vi "Dresden R2R Sputter 03.02.2018 IY24.vi"() -> ()   [LabVIEW 2009] (continued)
                                n30013 = Wait Until Next ms Multiple(millisecond multiple=u32 200) -> ()  [unwired: 1 out]
                                }
                                }
                                n30014 = local read "Semi"() -> (w34901:bool)
                                n30015 = Or(x=w34902, y=w34901) -> (x .or. y?=w34900:bool)
                                }
                                }
                                frame #1 {
                                }
                                }
                                }
                                frame #1 {
                                n30016 = local read "Semi"() -> (w34913:bool)
                                n30017 = case shown="False" w34913 {
                                frame #0 {
                                n30018 = local write "SDC1 10b"(TRUE ("SDC1 3")) -> ()
                                n30019 = Wait (ms)(milliseconds to wait=u32 1000) -> ()  [unwired: 1 out]
                                }
                                frame #1 {
                                }
                                }
                                }
                                }
                                }
                                frame #12 {
                                # "DC -Ignite Plasma"
                                n30020 = stacked-sequence {
                                frame #0 {
                                n30021 = local read "Semi"() -> (w34916:bool)
                                n30022 = case shown="False" w34916 {
                                frame #0 {
                                n30023 = stacked-sequence {
                                frame #0 {
                                n30024 = local read "Semi"() -> (w34917:bool)
                                n30025 = case shown="False" w34917 {
                                frame #0 {
                                n30026 = while {
                                i -> [w34923]
                                stop <- w34918 stop-if-true
                                n30027 = Greater?(x=w34923, y=50) -> (0:w34922:bool)
                                n30028 = case shown="True" w34922 {
                                frame #0 {
                                }
                                frame #1 {
                                n30029 = local write "Semi"(TRUE ("Semi")) -> ()
                                n30030 = local write "Error Message"("Sputtering Process cancelled.\nPlease check \nDC switch connections." ("Error Message")) -> ()
                                }
                                }
                                n30031 = local read "Cnt_Dcps_sw2_di"() -> (w34921:bool)
                                n30032 = case shown="False" w34921 {
                                tunnel: [FALSE ("Cnt_Dcps_sw1_do") TRUE ("Cnt_Dcps_sw1_do")] -> w34920
                                frame #0 {
                                n30033 = local write "Cnt_Dcps_sw2_do"(TRUE ("Cnt_Dcps_sw1_do")) -> ()
                                n30034 = Wait Until Next ms Multiple(millisecond multiple=u32 200) -> ()  [unwired: 1 out]
                                }
                                frame #1 {
                                }
                                }
                                n30035 = local read "Semi"() -> (w34919:bool)
                                n30036 = Or(x=w34920, y=w34919) -> (x .or. y?=w34918:bool)
                                }
                                }
                                frame #1 {
                                }
                                }
                                }
                                frame #1 {
                                n30037 = local read "Semi"() -> (w34931:bool)
                                n30038 = case shown="False" w34931 {
                                frame #0 {
                                n30039 = while {
                                i -> [w34937]
                                stop <- w34932 stop-if-true
                                n30040 = Greater?(x=w34937, y=50) -> (0:w34936:bool)
                                n30041 = case shown="True" w34936 {
                                frame #0 {
                                }
                                frame #1 {
                                n30042 = local write "Semi"(TRUE ("Semi")) -> ()
                                n30043 = local write "Error Message"("Sputtering Process cancelled.\nPlease check \nDC switch connections." ("Error Message")) -> ()
                                }
                                }
                                n30044 = local read "Cnt_Dcps_sw1_di"() -> (w34935:bool)
                                n30045 = case shown="True" w34935 {
                                tunnel: [TRUE ("Cnt_Dcps_sw1_do") FALSE ("Cnt_Dcps_sw1_do")] -> w34934
                                frame #0 {
                                }
                                frame #1 {
                                n30046 = local write "Cnt_Dcps_sw1_do"(FALSE ("Cnt_Dcps_sw1_do")) -> ()
                                n30047 = Wait Until Next ms Multiple(millisecond multiple=u32 200) -> ()  [unwired: 1 out]
                                }
                                }
                                n30048 = local read "Semi"() -> (w34933:bool)
                                n30049 = Or(x=w34934, y=w34933) -> (x .or. y?=w34932:bool)
                                }
                                }
                                frame #1 {
                                }
                                }
                                }
                                frame #2 {
                                n30050 = local read "Semi"() -> (w34945:bool)
                                n30051 = case shown="False" w34945 {
                                frame #0 {
                                n30052 = local write "Dc_host_auto"(TRUE ("Dc_host_auto")) -> ()
                                }
                                frame #1 {
                                }
                                }
                                }
                                frame #3 {
                                n30053 = local read "Semi"() -> (w34947:bool)
                                n30054 = case shown="False" w34947 {
                                frame #0 {
                                n30055 = local read "R Cmb Ch3 Step1 Coating Power"() -> (w34948:dbl)
                                n30056 = local write "Set DC Power       : 2"(w34948) -> ()
                                }
                                frame #1 {
                                }
                                }
                                }
                                frame #4 {
                                n30057 = local read "Semi"() -> (w34949:bool)
                                n30058 = case shown="False" w34949 {
                                frame #0 {
                                n30059 = Wait (ms)(milliseconds to wait=u32 1000) -> ()  [unwired: 1 out]
                                }
                                frame #1 {
                                }
                                }
                                }
                                frame #5 {
                                n30060 = local read "Semi"() -> (w34951:bool)
                                n30061 = case shown="False" w34951 {
                                frame #0 {
                                n30062 = local write "Dc_auto_set"(TRUE ("Dc_auto_set")) -> ()
                                }
                                frame #1 {
                                }
                                }
                                }
                                frame #6 {
                                n30063 = local read "Semi"() -> (w34953:bool)
                                n30064 = case shown="False" w34953 {
                                frame #0 {
                                n30065 = Wait (ms)(milliseconds to wait=u32 1000) -> ()  [unwired: 1 out]
                                }
                                frame #1 {
                                }
                                }
                                }
                                }
                                }
                                frame #1 {
                                }
                                }
                                }
                                frame #1 {
                                n30066 = local read "Semi"() -> (w34955:bool)
                                n30067 = case shown="False" w34955 {
                                frame #0 {
                                n30068 = Wait (ms)(milliseconds to wait=u32 1000) -> ()  [unwired: 1 out]
                                n30069 = local write "SDC1 13"(TRUE ("SDC1 13")) -> ()
                                }
                                frame #1 {
                                }
                                }
                                }
                                }
                                }
                                frame #13 {
                                n30070 = stacked-sequence {
                                frame #0 {
                                n30071 = local read "R Maximum diameter"() -> (w34959:dbl)
                                n30072 = local read "R Web speed(cm/min)"() -> (w34961:dbl)
                                n30073 = local read "R Minimum diameter"() -> (w34958:dbl)
                                n30074 = local read "R Web thicness"() -> (w34960:dbl)
                                n30075 = Wait (ms)(milliseconds to wait=u32 1000) -> ()  [unwired: 1 out]
                                n30076 = local write "Initial Min Diameter"(w34958) -> ()
                                n30077 = local write "Max Diameter"(w34959) -> ()
                                n30078 = local write "Web Thickness"(w34960) -> ()
                                n30079 = local write "Web Speed"(w34961) -> ()
                                }
                                frame #1 {
                                n30080 = local read "R Cmb Ch2 Step1 Coating Power Active"() -> (w34976:bool)
                                n30081 = local read "R Cmb Ch2 Step2 Coating Power Active"() -> (w34975:bool)
                                n30082 = local read "R Cmb Ch2 Step3 Coating Power Active"() -> (w34974:bool)
                                n30083 = local read "R Cmb Ch2 Step4 Coating Power Active"() -> (w34973:bool)
                                n30084 = local read "R Cmb Ch2 Step5 Coating Power Active"() -> (w34972:bool)
                                n30085 = Boolean To (0,1)(Boolean=w34976) -> (0, 1=w34971:i16)
                                n30086 = Boolean To (0,1)(Boolean=w34975) -> (0, 1=w34970:i16)
                                n30087 = Boolean To (0,1)(Boolean=w34974) -> (0, 1=w34969:i16)
                                n30088 = Boolean To (0,1)(Boolean=w34973) -> (0, 1=w34968:i16)
                                n30089 = Boolean To (0,1)(Boolean=w34972) -> (0, 1=w34967:i16)
                                n30090 = Compound Arithmetic op=ADD(w34971, w34970, w34969, w34968, w34967) -> (w34965:i16)
                                n30091 = local read "R Cmb Interval length"() -> (w34966:dbl)
                                n30092 = Wait (ms)(milliseconds to wait=u32 200) -> ()  [unwired: 1 out]
                                n30093 = Multiply(x=w34966, y=w34965) -> (x*y=w34964:dbl)
                                n30094 = local write "Total length"(w34964) -> ()
                                }
                                frame #2 {
                                n30095 = local write "Calculate 2"(TRUE ("Calculate_auto")) -> ()
                                }
                                frame #3 {
                                n30096 = Wait (ms)(milliseconds to wait=u32 100) -> ()  [unwired: 1 out]
                                n30097 = local write "Roll_side_select"(enum32{"Left to Right", "Right to Left"}."Left to Right" ("Roll_side_select")) -> ()
                                }
                                frame #4 {
                                n30098 = Wait (ms)(milliseconds to wait=u32 100) -> ()  [unwired: 1 out]
                                n30099 = local write "Parameters_auto_set"(TRUE ("Parameters_auto_set")) -> ()
                                }
                                frame #5 {
                                n30100 = while {
                                i -> [w34986]
                                stop <- w34982 stop-if-true
                                n30101 = Wait Until Next ms Multiple(millisecond multiple=u32 300) -> ()  [unwired: 1 out]
                                n30102 = Greater?(x=w34986, y=100) -> (0:w34983:bool)
                                n30103 = local read "Parameters_auto_set"() -> (w34987:bool)
                                n30104 = case shown="False" w34987 {
                                tunnel: [TRUE FALSE] -> w34984
                                frame #0 {
                                }
                                frame #1 {
                                }
                                }
                                n30105 = Or(x=w34984, y=w34983) -> (x .or. y?=w34982:bool)
                                }
                                }
                                frame #6 {
                                n30106 = local read "R Tension Value"() -> (w34991:dbl)
                                n30107 = Wait (ms)(milliseconds to wait=u32 200) -> ()  [unwired: 1 out]
                                n30108 = local write "TC1_set_value"(w34991) -> ()
                                }
                                frame #7 {
                                n30109 = local write "TC1_auto_set"(TRUE ("TC1_auto_set")) -> ()
                                }
                                frame #8 {
                                w34995 = u16 2 items=["1", "2", "3", "4"] ("Target Chamber Sensor")
                                n30110 = local write "Target Chamber Sensor"(w34995) -> ()
                                n30111 = Wait (ms)(milliseconds to wait=u32 200) -> ()  [unwired: 1 out]
                                }
                                frame #9 {
                                n30112 = local read "Total length"() -> (w34997:dbl)
                                n30113 = Wait (ms)(milliseconds to wait=u32 100) -> ()  [unwired: 1 out]
                                n30114 = local write "Region"(w34997) -> ()
                                }
                                frame #10 {
                                n30115 = local read "Semi"() -> (w34998:bool)
                                n30116 = case shown="False" w34998 {
                                frame #0 {
                                n30117 = stacked-sequence {
                                frame #0 {
                                # "Gas Flow"
                                n30118 = stacked-sequence {
                                frame #0 {
                                n30119 = local read "Semi"() -> (w34999:bool)
                                n30120 = case shown="False" w34999 {
                                frame #0 {
                                n30121 = stacked-sequence {
                                frame #0 {
                                n30122 = local read "Semi"() -> (w35000:bool)
                                n30123 = case shown="False" w35000 {
                                frame #0 {
                                n30124 = local read "R Argon Flow sccm"() -> (w35001:dbl)
                                n30125 = local write "Ar_sccm3_4"(w35001) -> ()
                                }
                                frame #1 {
                                }
                                }
                                }
                                frame #1 {
                                n30126 = local read "Semi"() -> (w35002:bool)
                                n30127 = case shown="False" w35002 {
                                frame #0 {
                                n30128 = local write "Mfc2_Ar _3_4_set"(TRUE ("Mfc_Ar _1_2_set")) -> ()
                                }
                                frame #1 {
                                }
                                }
                                }
                                frame #2 {
                                n30129 = local read "Semi"() -> (w35004:bool)
                                n30130 = case shown="False" w35004 {
                                frame #0 {
                                n30131 = while {
                                i -> [w35007]
                                stop <- w35009 stop-if-true
                                n30132 = Greater?(x=w35007, y=50) -> (0:w35006:bool)
                                n30133 = local read "Semi"() -> (w35005:bool)
                                n30134 = Or(x=w35005, y=w35006) -> (x .or. y?=w35009:bool)
                                }
                                }
                                frame #1 {
                                }
                                }
                                }
                                frame #3 {
                                n30135 = local read "Semi"() -> (w35010:bool)
                                n30136 = case shown="False" w35010 {
                                frame #0 {
                                n30137 = local read "Ar_sccm_act 2"() -> (w35011:dbl)
                                n30138 = Greater?(x=w35011, y=1) -> (0:w35012:bool)
                                n30139 = case shown="False" w35012 {
                                frame #0 {
                                n30140 = local read "R Argon Flow sccm"() -> (w35014:dbl)
                                n30141 = local write "Ar_sccm3_4"(w35014) -> ()
                                }
                                frame #1 {
                                }
                                }
                                }
                                frame #1 {
                                }
                                }
                                }
                                frame #4 {
                                n30142 = local read "Semi"() -> (w35015:bool)
                                n30143 = case shown="False" w35015 {
                                frame #0 {
                                n30144 = local read "Ar_sccm_act 2"() -> (w35016:dbl)
                                n30145 = Greater?(x=w35016, y=1) -> (0:w35017:bool)
                                n30146 = case shown="False" w35017 {
                                frame #0 {
                                n30147 = while {
                                i -> [w35020]
                                stop <- w35024 stop-if-true
                                n30148 = Greater?(x=w35020, y=50) -> (0:w35019:bool)
                                n30149 = local read "Semi"() -> (w35023:bool)
                                n30150 = case shown="False" w35023 {
                                tunnel: [FALSE TRUE] -> w35022
                                frame #0 {
                                n30151 = Wait Until Next ms Multiple(millisecond multiple=u32 200) -> ()  [unwired: 1 out]
                                }
                                frame #1 {
                                }
                                }
                                n30152 = Or(x=w35022, y=w35019) -> (x .or. y?=w35024:bool)
                                }
                                }
                                frame #1 {
                                }
                                }
                                }
                                frame #1 {
                                }
                                }
                                }
                                frame #5 {
                                n30153 = local read "Semi"() -> (w35028:bool)
                                n30154 = case shown="False" w35028 {
                                frame #0 {
                                n30155 = local read "Ar_sccm_act 2"() -> (w35029:dbl)
                                n30156 = Greater?(x=w35029, y=1) -> (0:w35030:bool)
                                n30157 = case shown="False" w35030 {
                                frame #0 {
                                n30158 = local write "Semi"(TRUE ("Semi")) -> ()
                                n30159 = local write "Error Message"("Coating process cancelled.\nPlease check connections." ("Error Message")) -> ()
                                }
                                frame #1 {
                                }
                                }
                                }
                                frame #1 {
                                }
                                }
                                }
                                }
                                }
                                frame #1 {
                                }
                                }
                                }
                                frame #1 {
                                n30160 = local read "Semi"() -> (w35034:bool)
                                n30161 = case shown="False" w35034 {
                                frame #0 {
                                n30162 = local write "SDC1 11"(TRUE ("SDC1 11")) -> ()
                                n30163 = Wait (ms)(milliseconds to wait=u32 1000) -> ()  [unwired: 1 out]
                                }
                                frame #1 {
                                }
                                }
                                }
                                }
                                }
                                frame #1 {
                                # "Set Pressure for ignite plasma"
                                n30164 = stacked-sequence {
                                frame #0 {
                                n30165 = local read "Semi"() -> (w35037:bool)
                                n30166 = case shown="False" w35037 {
                                frame #0 {
                                n30167 = stacked-sequence {
                                frame #0 {
                                n30168 = local read "Semi"() -> (w35038:bool)
                                n30169 = case shown="False" w35038 {
                                frame #0 {
                                n30170 = local write "Set_pressure_value 3"(10.0 ("Set_pressure_value 2")) -> ()
                                }
                                frame #1 {
                                }
                                }
                                }
                                frame #1 {
                                n30171 = local read "Semi"() -> (w35040:bool)
                                n30172 = case shown="False" w35040 {
                                frame #0 {
                                n30173 = Wait (ms)(milliseconds to wait=u32 1000) -> ()  [unwired: 1 out]
                                }
                                frame #1 {
                                }
                                }
                                }
                                frame #2 {
                                n30174 = local read "Semi"() -> (w35042:bool)
                                n30175 = case shown="False" w35042 {
                                frame #0 {
                                n30176 = local write "Pc_bv3_auto_set_pressure"(TRUE ("Pc_bv1_auto_set_pressure")) -> ()
                                }
                                frame #1 {
                                }
                                }
                                }
                                frame #3 {
                                n30177 = local read "Semi"() -> (w35044:bool)
                                n30178 = case shown="False" w35044 {
                                frame #0 {
                                n30179 = while {
                                i -> [w35055]
                                stop <- w35047 stop-if-true
                                w35045 = 10.0 ("Set_pressure_value 2")
                                n30180 = Greater?(x=w35055, y=300) -> (0:w35049:bool)
                                n30181 = Add(x=1.0, y=w35045) -> (x+y=w35051:dbl)
                                n30182 = Subtract(x=w35045, y=1.0) -> (x-y=w35052:dbl)
                                n30183 = local read "Pressure_ch3"() -> (w35046:i32)
                                n30184 = In Range and Coerce(upper limit=w35051, x=w35046, lower limit=w35052) -> (In Range?=w35050:bool)  [unwired: 1 out]
                                n30185 = case shown="False" w35050 {
                                tunnel: [FALSE TRUE] -> w35048
                                frame #0 {
                                n30186 = Wait Until Next ms Multiple(millisecond multiple=u32 200) -> ()  [unwired: 1 out]
                                }
                                frame #1 {
                                }
                                }
                                n30187 = Or(x=w35048, y=w35049) -> (x .or. y?=w35047:bool)
                                }
                                }
                                frame #1 {
                                }
                                }
                                }
                                frame #4 {
                                n30188 = local read "Semi"() -> (w35060:bool)
                                n30189 = case shown="False" w35060 {
                                frame #0 {
                                w35061 = 10.0 ("Set_pressure_value 2")
                                n30190 = Add(x=1.0, y=w35061) -> (x+y=w35064:dbl)
                                n30191 = Subtract(x=w35061, y=1.0) -> (x-y=w35065:dbl)
                                n30192 = local read "Pressure_ch3"() -> (w35062:i32)
                                n30193 = In Range and Coerce(upper limit=w35064, x=w35062, lower limit=w35065) -> (In Range?=w35063:bool)  [unwired: 1 out]
                                n30194 = case shown="False" w35063 {
                                frame #0 {
                                n30195 = local read "R Set Pressure mtorr"() -> (w35068:dbl)
                                n30196 = local write "Set_pressure_value 3"(w35068) -> ()
                                }
                                frame #1 {
                                }
                                }
                                }
                                frame #1 {
                                }
                                }
                                }
                                frame #5 {
                                n30197 = local read "Semi"() -> (w35069:bool)
                                n30198 = case shown="False" w35069 {
                                frame #0 {
                                w35070 = 10.0 ("Set_pressure_value 2")
                                n30199 = Add(x=1.0, y=w35070) -> (x+y=w35073:dbl)
                                n30200 = Subtract(x=w35070, y=1.0) -> (x-y=w35074:dbl)
                                n30201 = local read "Pressure_ch3"() -> (w35071:i32)
                                n30202 = In Range and Coerce(upper limit=w35073, x=w35071, lower limit=w35074) -> (In Range?=w35072:bool)  [unwired: 1 out]
                                n30203 = case shown="False" w35072 {
                                frame #0 {
                                n30204 = local write "Pc_bv3_auto_set_pressure"(TRUE ("Pc_bv1_auto_set_pressure")) -> ()
                                }
                                frame #1 {
                                }
                                }
                                }
                                frame #1 {
                                }
                                }
                                }
                                frame #6 {
                                n30205 = local read "Semi"() -> (w35078:bool)
                                n30206 = case shown="False" w35078 {
                                frame #0 {
                                n30207 = while {
                                i -> [w35089]
                                stop <- w35081 stop-if-true
                                w35079 = 10.0 ("Set_pressure_value 2")
                                n30208 = Greater?(x=w35089, y=300) -> (0:w35083:bool)
                                n30209 = Add(x=1.0, y=w35079) -> (x+y=w35085:dbl)
                                n30210 = Subtract(x=w35079, y=1.0) -> (x-y=w35086:dbl)
                                n30211 = local read "Pressure_ch3"() -> (w35080:i32)
                                n30212 = In Range and Coerce(upper limit=w35085, x=w35080, lower limit=w35086) -> (In Range?=w35084:bool)  [unwired: 1 out]
                                n30213 = case shown="False" w35084 {
                                tunnel: [FALSE TRUE] -> w35082
                                frame #0 {
                                n30214 = Wait Until Next ms Multiple(millisecond multiple=u32 200) -> ()  [unwired: 1 out]
                                }
                                frame #1 {
                                }
                                }
                                n30215 = Or(x=w35082, y=w35083) -> (x .or. y?=w35081:bool)
                                }
                                }
                                frame #1 {
                                }
                                }
                                }
                                frame #7 {
                                n30216 = local read "Semi"() -> (w35094:bool)
                                n30217 = case shown="False" w35094 {
                                frame #0 {
                                n30218 = local read "Set_pressure_value 3"() -> (w35097:dbl)
                                n30219 = Add(x=1.0, y=w35097) -> (x+y=w35098:dbl)
                                n30220 = Subtract(x=w35097, y=1.0) -> (x-y=w35099:dbl)
                                n30221 = local read "Pressure_ch3"() -> (w35095:i32)
                                n30222 = In Range and Coerce(upper limit=w35098, x=w35095, lower limit=w35099) -> (In Range?=w35096:bool)  [unwired: 1 out]
                                n30223 = case shown="False" w35096 {
                                frame #0 {
                                n30224 = local write "Semi"(TRUE ("Semi")) -> ()
                                n30225 = local write "Error Message"("Coating Pressure could not be adjusted !" ("Error Message")) -> ()
                                }
                                frame #1 {
                                }
                                }
                                }
                                frame #1 {
                                }
                                }
                                }
                                }
                                }
                                frame #1 {
                                }
                                }
                                }
                                frame #1 {
                                n30226 = local read "Semi"() -> (w35104:bool)
                                n30227 = case shown="False" w35104 {
                                frame #0 {
                                n30228 = local write "SDC1 9"(TRUE ("SDC1 9")) -> ()
                                n30229 = Wait (ms)(milliseconds to wait=u32 1000) -> ()  [unwired: 1 out]
                                }
                                frame #1 {
                                }
                                }
                                }
                                }
                                }
                                frame #2 {
                                # "Plasma ignite and check"
                                n30230 = stacked-sequence {
                                frame #0 {
                                n30231 = local read "Semi"() -> (w35107:bool)
                                n30232 = case shown="False" w35107 {
                                frame #0 {
                                n30233 = local write "Dc_auto_on"(TRUE ("Dc_auto_on")) -> ()
                                }
                                frame #1 {
                                }
                                }
                                }
                                frame #1 {
                                n30234 = local read "Semi"() -> (w35109:bool)
                                n30235 = case shown="False" w35109 {
                                frame #0 {
                                n30236 = while {
                                i -> [w35119]
                                stop <- w35110 stop-if-true
                                n30237 = Greater Or Equal?(x=w35119, y=240) -> (x >= y?=w35118:bool)
                                n30238 = case shown="True" w35118 {
                                frame #0 {
                                }
                                frame #1 {
                                n30239 = local write "Semi"(TRUE ("Semi")) -> ()
                                }
                                }
                                n30240 = local read "Set DC Power       : 2"() -> (w35115:dbl)
                                n30241 = local read "Actual DC Power : 2"() -> (w35114:dbl)
                                n30242 = Subtract(x=w35115, y=w35114) -> (x-y=w35117:dbl)
                                n30243 = Less?(x=w35117, y=10.0) -> (x < y?=w35112:bool)
                                n30244 = local read "Semi"() -> (w35111:bool)
                                n30245 = Or(x=w35112, y=w35111) -> (x .or. y?=w35110:bool)
                                n30246 = Wait Until Next ms Multiple(millisecond multiple=u32 500) -> ()  [unwired: 1 out]
                                }
                                }
                                frame #1 {
                                }
                                }
                                }
                                }
                                }
                                frame #3 {
                                # "Set Pressure for coating"
                                n30247 = stacked-sequence {
                                frame #0 {
                                n30248 = local read "Semi"() -> (w35122:bool)
                                n30249 = case shown="False" w35122 {
                                frame #0 {
                                n30250 = stacked-sequence {
                                frame #0 {
                                n30251 = local read "Semi"() -> (w35123:bool)
                                n30252 = case shown="False" w35123 {
                                frame #0 {
                                n30253 = local read "R Set Pressure mtorr"() -> (w35124:dbl)
                                n30254 = local write "Set_pressure_value 3"(w35124) -> ()
                                }
                                frame #1 {
                                }
                                }
                                }
                                frame #1 {
                                n30255 = local read "Semi"() -> (w35125:bool)
                                n30256 = case shown="False" w35125 {
                                frame #0 {
                                n30257 = Wait (ms)(milliseconds to wait=u32 200) -> ()  [unwired: 1 out]
                                }
                                frame #1 {
                                }
                                }
                                }
                                frame #2 {
                                n30258 = local read "Semi"() -> (w35127:bool)
                                n30259 = case shown="False" w35127 {
                                frame #0 {
                                n30260 = local write "Pc_bv3_auto_set_pressure"(TRUE ("Pc_bv1_auto_set_pressure")) -> ()
                                }
                                frame #1 {
                                }
                                }
                                }
                                frame #3 {
                                n30261 = local read "Semi"() -> (w35129:bool)
                                n30262 = case shown="False" w35129 {
                                frame #0 {
                                n30263 = while {
                                i -> [w35140]
                                stop <- w35132 stop-if-true
                                n30264 = local read "Set_pressure_value 3"() -> (w35130:dbl)
                                n30265 = Greater?(x=w35140, y=300) -> (0:w35134:bool)
                                n30266 = Add(x=1.0, y=w35130) -> (x+y=w35136:dbl)
                                n30267 = Subtract(x=w35130, y=1.0) -> (x-y=w35137:dbl)
                                n30268 = local read "Pressure_ch3"() -> (w35131:i32)
                                n30269 = In Range and Coerce(upper limit=w35136, x=w35131, lower limit=w35137) -> (In Range?=w35135:bool)  [unwired: 1 out]
                                n30270 = case shown="False" w35135 {
                                tunnel: [FALSE TRUE] -> w35133
                                frame #0 {
                                n30271 = Wait Until Next ms Multiple(millisecond multiple=u32 200) -> ()  [unwired: 1 out]
                                }
                                frame #1 {
                                }
                                }
                                n30272 = Or(x=w35133, y=w35134) -> (x .or. y?=w35132:bool)
                                }
                                }
                                frame #1 {
                                }
                                }
                                }
                                frame #4 {
                                n30273 = local read "Semi"() -> (w35145:bool)
                                n30274 = case shown="False" w35145 {
                                frame #0 {
                                n30275 = local read "Set_pressure_value 3"() -> (w35146:dbl)
                                n30276 = Add(x=1.0, y=w35146) -> (x+y=w35149:dbl)
                                n30277 = Subtract(x=w35146, y=1.0) -> (x-y=w35150:dbl)
                                n30278 = local read "Pressure_ch3"() -> (w35147:i32)
                                n30279 = In Range and Coerce(upper limit=w35149, x=w35147, lower limit=w35150) -> (In Range?=w35148:bool)  [unwired: 1 out]
                                n30280 = case shown="False" w35148 {
                                frame #0 {
                                n30281 = local read "R Set Pressure mtorr"() -> (w35153:dbl)
                                n30282 = local write "Set_pressure_value 3"(w35153) -> ()
                                }
                                frame #1 {
                                }
                                }
                                }
                                frame #1 {
                                }
                                }
                                }
                                frame #5 {
                                n30283 = local read "Semi"() -> (w35154:bool)
                                n30284 = case shown="False" w35154 {
                                frame #0 {
                                n30285 = local read "Set_pressure_value 3"() -> (w35155:dbl)
                                n30286 = Add(x=1.0, y=w35155) -> (x+y=w35158:dbl)
                                n30287 = Subtract(x=w35155, y=1.0) -> (x-y=w35159:dbl)
                                n30288 = local read "Pressure_ch3"() -> (w35156:i32)
                                n30289 = In Range and Coerce(upper limit=w35158, x=w35156, lower limit=w35159) -> (In Range?=w35157:bool)  [unwired: 1 out]
                                n30290 = case shown="False" w35157 {
                                frame #0 {
                                n30291 = local write "Pc_bv3_auto_set_pressure"(TRUE ("Pc_bv1_auto_set_pressure")) -> ()
                                }
                                frame #1 {
                                }
                                }
                                }
                                frame #1 {
                                }
                                }
                                }
                                frame #6 {
                                n30292 = local read "Semi"() -> (w35163:bool)
                                n30293 = case shown="False" w35163 {
                                frame #0 {
                                n30294 = while {
                                i -> [w35174]
                                stop <- w35165 stop-if-true
                                n30295 = local read "Set_pressure_value 3"() -> (w35169:dbl)
                                n30296 = Greater?(x=w35174, y=300) -> (0:w35167:bool)
                                n30297 = Add(x=1.0, y=w35169) -> (x+y=w35170:dbl)
                                n30298 = Subtract(x=w35169, y=1.0) -> (x-y=w35171:dbl)
                                n30299 = local read "Pressure_ch3"() -> (w35164:i32)
                                n30300 = In Range and Coerce(upper limit=w35170, x=w35164, lower limit=w35171) -> (In Range?=w35168:bool)  [unwired: 1 out]
                                n30301 = case shown="False" w35168 {
                                tunnel: [FALSE TRUE] -> w35166
                                frame #0 {
                                n30302 = Wait Until Next ms Multiple(millisecond multiple=u32 200) -> ()  [unwired: 1 out]
                                }
                                frame #1 {
                                }
                                }
                                n30303 = Or(x=w35166, y=w35167) -> (x .or. y?=w35165:bool)
                                }
                                }
                                frame #1 {
                                }
                                }
                                }
                                frame #7 {
                                n30304 = local read "Semi"() -> (w35179:bool)
                                n30305 = case shown="False" w35179 {
                                frame #0 {
                                n30306 = local read "Set_pressure_value 3"() -> (w35182:dbl)
                                n30307 = Add(x=1.0, y=w35182) -> (x+y=w35183:dbl)
                                n30308 = Subtract(x=w35182, y=1.0) -> (x-y=w35184:dbl)
                                n30309 = local read "Pressure_ch3"() -> (w35180:i32)
                                n30310 = In Range and Coerce(upper limit=w35183, x=w35180, lower limit=w35184) -> (In Range?=w35181:bool)  [unwired: 1 out]
                                n30311 = case shown="False" w35181 {
                                frame #0 {
                                n30312 = local write "Semi"(TRUE ("Semi")) -> ()
                                n30313 = local write "Error Message"("Coating Pressure could not be adjusted !" ("Error Message")) -> ()
                                }
                                frame #1 {
                                }
                                }
                                }
                                frame #1 {
                                }
                                }
                                }
                                }
                                }
                                frame #1 {
                                }
                                }
                                }
                                frame #1 {
                                n30314 = local read "Semi"() -> (w35189:bool)
                                n30315 = case shown="False" w35189 {